vi "UHR-Fleezers Control (host) - 12.7b.vi"() -> ()   [LabVIEW 2012] (continued)
                                frame #0 {
                                n1177 = property on="Trap Delta (MHz)" class="DigNum (strict)"("Val(Sgnl)"=w1735) -> ()  [unwired: 2 in, 2 out]
                                }
                                frame #1 {
                                n1178 = Wait (ms)(milliseconds to wait=u32 500) -> ()  [unwired: 1 out]
                                }
                                frame #2 {
                                n1179 = local read "Shift confocal"() -> (w1739:bool)
                                n1180 = local read "Mean"() -> (w1737:dbl)
                                n1181 = Greater?(x=w1737, y=11.0) -> (0:w1740:bool)
                                n1182 = Not(x=w1740) -> (.not. x?=w1741:bool)
                                n1183 = And(x=w1741, y=w1739) -> (x .and. y?=w1743:bool)
                                n1184 = And(x=w1740, y=w1739) -> (x .and. y?=w1742:bool)
                                n1185 = case shown="True" w1742 {
                                frame False {
                                }
                                frame True {
                                n1186 = local read "Confocal Y 2 (V)"() -> (w1747:dbl)
                                n1187 = local read "Confocal X 2 (V)"() -> (w1746:dbl)
                                n1188 = property on="AO1" class="Slide (strict)"("Val(Sgnl)"=w1747) -> ()  [unwired: 2 in, 2 out]
                                n1189 = property on="AO2" class="Slide (strict)"("Val(Sgnl)"=w1746) -> ()  [unwired: 2 in, 2 out]
                                }
                                }
                                n1190 = case shown="True" w1743 {
                                frame False {
                                }
                                frame True {
                                n1191 = local read "Confocal X 1 (V)"() -> (w1744:dbl)
                                n1192 = local read "Confocal Y 1 (V)"() -> (w1745:dbl)
                                n1193 = property on="AO2" class="Slide (strict)"("Val(Sgnl)"=w1744) -> ()  [unwired: 2 in, 2 out]
                                n1194 = property on="AO1" class="Slide (strict)"("Val(Sgnl)"=w1745) -> ()  [unwired: 2 in, 2 out]
                                }
                                }
                                }
                                }
                                }
                                }
                                }
                              }
                            }
                          }
                          n1195 = local read "Time (s)"() -> (w1681:dbl)
                          "Fl. High" <- TRUE ("Yanking")
                        }
                        frame #1 {
                          n1196 = local read "Auto F Reset"() -> (w1748:bool)
                          n1197 = case shown="True" w1748 {
                            tunnel: w1753 -> [_ w1757]
                            tunnel: w1752 -> [_ w1756]
                            tunnel: w1751 -> [_ w1755]
                            tunnel: w1749 -> [_ w1754]
                            frame False {
                            }
                            frame True {
                              n1198 = node-c288() -> (w1759:T23)  [unwired: 4 out]
                              n1199 = timed-loop {
                                timing: w1759 -> [_]
                                timing-out: [_] -> w1758
                                tunnel: w1757 -> [w1777]
                                tunnel: w1756 -> [w1776]
                                tunnel: w1755 -> [w1775]
                                tunnel: w1754 -> [w1774]
                                stop <- w1760 stop-if-true
                                n1200 = node-c288() -> ()  [unwired: 2 out]
                                n1201 = local read "Fl. Delta Thresh. (kHz)"() -> (w1768:dbl)
                                n1202 = local read "Fl. Triggered..."() -> (w1773:bool)
                                n1203 = local read "Delta Fl. 1"() -> (w1764:dbl)
                                n1204 = local read "Delta Fl. 2"() -> (w1762:dbl)
                                n1205 = local read "Stop All"() -> (w1771:bool)
                                n1206 = local read "APD to Watch"() -> (w1763:bool)
                                n1207 = Select(t=w1764, s=w1763, f=w1762) -> (s? t:f=w1761:dbl)
                                n1208 = Not(x=w1773) -> (.not. x?=w1772:bool)
                                n1209 = Multiply(x=w1768, y=1000.0) -> (x*y=w1767:dbl)
                                n1210 = Negate(x=w1767) -> (-x=w1766:dbl)
                                n1211 = Less?(x=w1761, y=w1766) -> (x < y?=w1770:bool)
                                n1212 = Compound Arithmetic op=OR(w1770, w1771, w1772, "Reset Force") -> (w1760:bool)
                                n1213 = case shown="True" w1760 {
                                tunnel: w1777 -> [_ w1792]
                                tunnel: w1776 -> [_ w1791]
                                tunnel: w1775 -> [_ w1781]
                                tunnel: w1774 -> [_ w1783]
                                frame False {
                                }
                                frame True {
                                n1214 = local read "Time (s)"() -> (w1782:dbl)
                                n1215 = case shown="\"Yank\"" w1791 {
                                tunnel: w1792 -> [_ w1795]
                                tunnel: w1783 -> [_ w1793]
                                frame "Image", Default {
                                }
                                frame "Yank" {
                                n1216 = flat-sequence {
                                tunnel: [w1801] -> w1796
                                tunnel: w1795 -> [w1801]
                                tunnel: [w1797] -> w1794
                                tunnel: w1793 -> [w1797]
                                tunnel: w1796 -> [w1804]
                                tunnel: w1794 -> [w1802]
                                frame #0 {
                                n1217 = local read "Yank Delay (s)"() -> (w1800:dbl)
                                n1218 = Multiply(x=w1800, y=1000.0) -> (x*y=w1798:dbl)
                                n1219 = Wait (ms)(milliseconds to wait=w1798) -> ()  [unwired: 1 out]
                                }
                                frame #1 {
                                n1220 = local read "Yank to which?"() -> (w1803:bool)
                                n1221 = case shown="False" w1803 {
                                tunnel: w1804 -> [_ w1831]
                                tunnel: w1802 -> [w1805 _]
                                frame False {
                                n1222 = flat-sequence {
                                tunnel: w1805 -> [w1806]
                                frame #0 {
                                n1223 = property on="Trap Pos FB SP" class="DigNum (strict)"("Val(Sgnl)"=w1806) -> ()  [unwired: 2 in, 2 out]
                                }
                                frame #1 {
                                n1224 = Wait (ms)(milliseconds to wait=u32 700) -> ()  [unwired: 1 out]
                                }
                                frame #2 {
                                n1225 = local read "Action (%)"() -> (w1811:dbl)
                                n1226 = Absolute Value(x=w1811) -> (abs(x)=w1810:dbl)
                                n1227 = Greater?(x=w1810, y=70.0) -> (0:w1808:bool)
                                n1228 = property on="Remove Action Offset" class="Bool (strict)"("Val(Sgnl)"=w1808) -> ()  [unwired: 2 in, 2 out]
                                }
                                frame #3 {
                                n1229 = for {
                                N: 4 -> [_]
                                n1230 = flat-sequence {
                                frame #0 {
                                n1231 = Wait (ms)(milliseconds to wait=u32 500) -> ()  [unwired: 1 out]
                                }
                                frame #1 {
                                n1232 = local read "Action (%)"() -> (w1817:dbl)
                                n1233 = Absolute Value(x=w1817) -> (abs(x)=w1816:dbl)
                                n1234 = Greater?(x=w1816, y=70.0) -> (0:w1814:bool)
                                n1235 = property on="Remove Action Offset" class="Bool (strict)"("Val(Sgnl)"=w1814) -> ()  [unwired: 2 in, 2 out]
                                }
                                }
                                }
                                }
                                frame #4 {
                                n1236 = local read "Shift confocal"() -> (w1822:bool)
                                n1237 = local read "Mean"() -> (w1824:dbl)
                                n1238 = Greater?(x=w1824, y=11.0) -> (0:w1821:bool)
                                n1239 = Not(x=w1821) -> (.not. x?=w1820:bool)
                                n1240 = And(x=w1821, y=w1822) -> (x .and. y?=w1819:bool)
                                n1241 = And(x=w1820, y=w1822) -> (x .and. y?=w1818:bool)
                                n1242 = case shown="True" w1819 {
                                frame False {
                                }
                                frame True {
                                n1243 = local read "Confocal Y 2 (V)"() -> (w1828:dbl)
                                n1244 = local read "Confocal X 2 (V)"() -> (w1827:dbl)
                                n1245 = property on="AO2" class="Slide (strict)"("Val(Sgnl)"=w1827) -> ()  [unwired: 2 in, 2 out]
                                n1246 = property on="AO1" class="Slide (strict)"("Val(Sgnl)"=w1828) -> ()  [unwired: 2 in, 2 out]
                                }
                                }
                                n1247 = case shown="True" w1818 {
                                frame False {
                                }
                                frame True {
                                n1248 = local read "Confocal X 1 (V)"() -> (w1825:dbl)
                                n1249 = local read "Confocal Y 1 (V)"() -> (w1826:dbl)
                                n1250 = property on="AO1" class="Slide (strict)"("Val(Sgnl)"=w1826) -> ()  [unwired: 2 in, 2 out]
                                n1251 = property on="AO2" class="Slide (strict)"("Val(Sgnl)"=w1825) -> ()  [unwired: 2 in, 2 out]
                                }
                                }
                                }
                                frame #5 {
                                n1252 = Wait (ms)(milliseconds to wait=u32 1500) -> ()  [unwired: 1 out]
                                }
                                frame #6 {
                                n1253 = property on="Rem fb disp offset" class="Bool (strict)"("Val(Sgnl)"=TRUE ("Value (Signaling)")) -> ()  [unwired: 2 in, 2 out]
                                }
                                }
                                }
                                frame True {
                                n1254 = flat-sequence {
                                tunnel: w1831 -> [w1832]
                                frame #0 {
                                n1255 = property on="Trap Delta (MHz)" class="DigNum (strict)"("Val(Sgnl)"=w1832) -> ()  [unwired: 2 in, 2 out]
                                }
                                frame #1 {
                                n1256 = Wait (ms)(milliseconds to wait=u32 500) -> ()  [unwired: 1 out]
                                }
                                frame #2 {
                                n1257 = local read "Shift confocal"() -> (w1838:bool)
                                n1258 = local read "Mean"() -> (w1840:dbl)
                                n1259 = Greater?(x=w1840, y=11.0) -> (0:w1837:bool)
                                n1260 = Not(x=w1837) -> (.not. x?=w1836:bool)
                                n1261 = And(x=w1837, y=w1838) -> (x .and. y?=w1835:bool)
                                n1262 = And(x=w1836, y=w1838) -> (x .and. y?=w1834:bool)
                                n1263 = case shown="True" w1835 {
                                frame False {
                                }
                                frame True {
                                n1264 = local read "Confocal Y 2 (V)"() -> (w1844:dbl)
                                n1265 = local read "Confocal X 2 (V)"() -> (w1843:dbl)
                                n1266 = property on="AO2" class="Slide (strict)"("Val(Sgnl)"=w1843) -> ()  [unwired: 2 in, 2 out]
                                n1267 = property on="AO1" class="Slide (strict)"("Val(Sgnl)"=w1844) -> ()  [unwired: 2 in, 2 out]
                                }
                                }
                                n1268 = case shown="True" w1834 {
                                frame False {
                                }
                                frame True {
                                n1269 = local read "Confocal Y 1 (V)"() -> (w1842:dbl)
                                n1270 = local read "Confocal X 1 (V)"() -> (w1841:dbl)
                                n1271 = property on="AO2" class="Slide (strict)"("Val(Sgnl)"=w1841) -> ()  [unwired: 2 in, 2 out]
                                n1272 = property on="AO1" class="Slide (strict)"("Val(Sgnl)"=w1842) -> ()  [unwired: 2 in, 2 out]
                                }
                                }
                                }
                                }
                                }
                                }
                                }
                                }
                                }
                                }
                                n1273 = local read "Messages"() -> (w1790:string)
                                n1274 = Subtract(x=w1782, y=w1781) -> (x-y=w1788:dbl)
                                "Duration (s)" <- w1788
                                n1275 = Number To Decimal String(number=w1788, width (-)=i16 0) -> (decimal integer string=w1786:string)
                                n1276 = Concatenate Strings(w1786, " s fluorescence event." ("string")) -> (w1784:string)
                                n1277 = call "Update messages.vi"("Message to add"=w1784, "Old message string"=w1790) -> ("New message string"=w1789:string)
                                n1278 = local write "Reset Force"(FALSE ("Reset Force")) -> ()
                                n1279 = local write "Waiting"(TRUE ("Waiting")) -> ()
                                n1280 = local write "Messages"(w1789) -> ()
                                n1281 = local write "Fl. High"(FALSE ("Fl. High")) -> ()
                                n1282 = call <vilib>:"Beep.vi"() -> ()  [unwired: 3 in, 9 out]
                                }
                                }
                                n1283 = node-c288() -> ()  [unwired: 2 out]
                              }
                              n1284 = node-c288(w1758) -> ()  [unwired: 1 out]
                            }
                          }
                        }
                      }
                      n1285 = local read "Trap Delta (MHz)"() -> (w1673:dbl)
                      n1286 = local read "Trap Pos FB SP"() -> (w1668:fxp<+/-,16,1>)
                    }
                  }
                }
                frame #1 {
                  n1287 = local read "Stop All"() -> (w1854:bool)
                  n1288 = local read "Fl. Triggered..."() -> (w1852:bool)
                  n1289 = Not(x=w1852) -> (.not. x?=w1853:bool)
                  n1290 = Or(x=w1853, y=w1854) -> (x .or. y?=w1851:bool)
                }
              }
              n1291 = case shown="True" w1445 {
                frame False {
                }
                frame True {
                  n1292 = local read "Confocal Y 1 (V)"() -> (w1455:dbl)
                  n1293 = local read "Confocal X 1 (V)"() -> (w1454:dbl)
                  n1294 = property on="AO2" class="Slide (strict)"("Val(Sgnl)"=w1454) -> ()  [unwired: 2 in, 2 out]
                  n1295 = property on="AO1" class="Slide (strict)"("Val(Sgnl)"=w1455) -> ()  [unwired: 2 in, 2 out]
                }
              }
              n1296 = case shown="True" w1445 {
                frame False {
                }
                frame True {
                  w1453 = FALSE ("Fl. High")
                  n1297 = local write "Waiting"(w1453) -> ()
                  n1298 = local write "Fl. High"(w1453) -> ()
                }
              }
              n1299 = node-c288() -> ()  [unwired: 2 out]
            }
            n1300 = node-c288(w1443) -> ()  [unwired: 1 out]
          }
        }
      }
      event "Stop All": Value Change {
        n1301 = event-data() -> ()  [unwired: 7 out]
        n1302 = local read "Stop All"() -> (w1859:bool)
      }
    }
    n1303 = node-c288() -> ()  [unwired: 2 out]
  }
  n1304 = timed-loop "Basic control parameters (all FPGA settings, other basic controls)" {
    tunnel: w23 -> [w1868]
    shift-right: [w1867] -> _
    shift-left: errorcluster {"status"=FALSE, "code"=0, "source"=""} ("error out") -> [w1866]
    tunnel: [w1865] -> _
    timing: w133 -> [_]
    timing-out: [_] -> w132
    tunnel: w106 -> [w1864]
    tunnel: w78 -> [w1863]
    tunnel: w77 -> [w1862]
    tunnel: w76 -> [w1861]
    tunnel: w75 -> [w1860]
    stop <- w1865 stop-if-true
    n1305 = node-c288() -> ()  [unwired: 2 out]
    n1306 = event shown="[14] \"DIO count 1 (ticks)\", \"DIO count 2 (ticks)\", \"DIO count 3 (ticks)\", \"Interlace\", \"Number Interlace Sets\", \"Not-Interlacing Set\", \"BD 1 Delay (ticks)\", \"BD 2 Delay (Ticks)\", \"Next trap write delay (ticks)\", \"XY phase ext loop method\", \"Amp switch delay 2\", \"BD 2 Delay (Ticks) 2\", \"BD 1 Delay (ticks) 2\": Value Change" {
      selector: _ -> [_ _ _ _ _ _ _ _ _ _ _ _ _ _ _ _ _ _ _ _ _ _ _ _ _ _ _ _ _ _ _ _ _ _ _ _ _ _ _ _ _ _ _ _ _ _ _ _ _ _ _ _ _ _ _ _ _ _ _ _ _ _ _ _ _ _ _ _ _ _ _ _ _ _]
      dyn-events: _ -> [_ _ _ _ _ _ _ _ _ _ _ _ _ _ _ _ _ _ _ _ _ _ _ _ _ _ _ _ _ _ _ _ _ _ _ _ _ _ _ _ _ _ _ _ _ _ _ _ _ _ _ _ _ _ _ _ _ _ _ _ _ _ _ _ _ _ _ _ _ _ _ _ _ _]
      timeout: _ -> [_ _ _ _ _ _ _ _ _ _ _ _ _ _ _ _ _ _ _ _ _ _ _ _ _ _ _ _ _ _ _ _ _ _ _ _ _ _ _ _ _ _ _ _ _ _ _ _ _ _ _ _ _ _ _ _ _ _ _ _ _ _ _ _ _ _ _ _ _ _ _ _ _ _]
      tunnel: w1868 -> [w1909 _ _ _ w1947 _ w1969 _ _ _ _ w2035 _ _ w2085 w2091 w2098 w2103 w2176 _ w2192 w2217 w2238 w2259 w2279 w2308 w2334 w2337 w2341 w2436 w2441 w2479 _ w2514 w2518 w2529 w2533 w2537 _ w2545 _ _ _ _ _ _ _ _ _ _ _ _ _ _ _ _ _ w2923 _ w2940 _ w2947 w2965 _ w2972 w2980 w2995 w3011 w3017 _ w3026 _ w3045 _]
      tunnel: [w1908 _ _ _ w1937 _ w1968 _ _ w2000 _ w2014 _ _ w2084 w2087 w2097 w2100 w2170 _ w2191 w2216 w2236 w2257 w2277 w2302 w2332 _ w2339 w2434 w2439 w2477 _ w2512 w2516 w2520 w2531 w2535 _ w2543 _ _ _ _ _ _ _ _ _ _ _ _ _ _ _ _ _ w2921 _ _ _ _ w2962 _ _ _ _ _ _ _ _ _ _ _] -> w1867
      tunnel: w1866 -> [w1907 _ _ _ w1946 _ w1967 _ _ w2000 _ w2034 _ _ w2083 w2086 w2096 w2099 w2175 _ w2190 w2215 w2237 w2258 w2278 w2307 w2333 w2336 w2340 w2435 w2440 w2478 _ w2513 w2517 w2528 w2532 w2536 _ w2544 _ _ _ _ _ _ _ _ _ _ _ _ _ _ _ _ _ w2922 _ w2939 _ w2946 w2964 _ w2971 w2979 w2994 w3010 w3016 _ w3025 _ w3044 _]
      tunnel: [_ _ _ _ _ _ _ _ _ w1999 _ _ _ _ _ _ _ _ _ _ _ _ _ _ _ _ _ _ _ _ _ _ _ _ _ _ _ _ _ _ _ _ _ _ _ _ _ _ _ _ _ _ _ _ _ _ _ _ _ _ _ _ _ _ _ _ _ _ _ _ _ _ _ _] -> w1865
      tunnel: [_ _ _ _ _ _ _ "Round T1 X" _ _ _ _ _ _ _ _ _ _ _ _ _ _ _ _ _ _ _ _ _ _ _ _ _ _ _ _ _ _ _ _ _ _ _ _ _ _ _ _ _ _ _ _ _ _ _ _ _ _ _ _ _ _ _ _ _ _ _ _ _ _ _ _ _ _] -> _
      tunnel: [_ _ _ "Adjust Scale\nto Mean" _ _ _ _ _ _ _ _ _ _ _ _ _ _ _ _ _ _ _ _ _ _ _ _ "Test ttrig" _ _ _ _ _ _ _ _ _ _ _ _ _ _ _ _ _ _ "Flush Sample" "Flush Pump 3" "Flush Pump 1" "Clear Volume" _ _ _ _ _ _ _ _ _ _ _ _ _ _ _ _ _ _ _ _ _ _ _] -> _
      tunnel: [_ _ _ _ _ _ _ _ "Round T2 X" _ "Delayed Interlace Start" _ _ _ _ _ _ _ _ _ _ _ _ _ _ _ _ _ _ _ _ _ _ _ _ _ _ _ _ _ _ _ _ _ _ _ _ _ _ _ _ _ _ _ _ _ _ _ _ _ _ _ _ _ _ _ _ _ _ _ _ _ _ _] -> _
      tunnel: w1864 -> [_ _ _ _ _ _ _ _ _ _ _ _ _ _ _ _ _ _ _ _ _ _ _ _ _ _ _ _ _ _ _ _ _ _ _ _ _ _ _ _ _ _ _ w2702 w2709 w2716 w2721 w2730 _ _ w2836 _ _ _ _ _ _ _ _ _ _ _ _ _ _ _ _ _ _ _ _ _ _ _]
      tunnel: w1863 -> [_ _ _ _ _ _ _ _ _ _ _ _ _ _ _ _ _ _ _ _ _ _ _ _ _ _ _ _ _ _ _ _ _ _ _ _ _ _ _ _ _ w2619 _ _ _ _ _ _ w2774 _ _ w2842 _ w2851 _ w2865 _ _ _ _ _ _ _ _ _ _ _ _ _ _ _ _ _ _]
      tunnel: w1862 -> [_ _ _ _ _ _ _ _ _ _ _ _ _ _ _ _ _ _ _ _ _ _ _ _ _ _ _ _ _ _ _ _ _ _ _ _ _ _ _ _ _ _ _ _ _ _ _ _ _ _ _ _ _ _ _ _ _ _ _ _ _ _ _ _ _ _ _ _ _ _ _ _ _ _]
      tunnel: w1861 -> [_ _ _ _ _ _ _ _ _ _ _ _ _ _ _ _ _ _ _ _ _ _ _ _ _ _ _ _ _ _ _ _ _ _ _ _ _ _ _ _ w2556 _ _ _ _ _ _ _ _ w2804 _ _ w2847 _ w2858 _ w2890 _ _ _ _ _ _ _ _ _ _ _ _ _ _ _ _ _]
      tunnel: w1860 -> [_ _ _ _ _ _ _ _ _ _ _ _ _ _ _ _ _ _ _ _ _ _ _ _ _ _ _ _ _ _ _ _ _ _ _ _ _ _ _ _ _ _ _ _ _ _ _ _ _ _ _ _ _ _ _ _ _ _ _ _ _ _ _ _ _ _ _ _ _ _ _ _ _ _]
      event "AI Count (ticks)", "Sets to FIFO (Traps)", "Save ave N", "FPGA Ave.", "# Samples/channel", "N sets to save": Value Change {
        # "So that if 'Save ave N' is updated, the AOD scanning code updates too."
        n1307 = event-data() -> ()  [unwired: 6 out]
        n1308 = local read "AI Count (ticks)"() -> (w1891:u16)
        n1309 = Unbundle By Name("Sets to FIFO (Traps)") -> ("Set 1"=w1874:bool, "Set 2"=w1873:bool, "Set 3"=w1872:bool)
        n1310 = Boolean To (0,1)(Boolean="Sets to FIFO (Traps)") -> (0, 1=w1899:cluster{"Set 1":i16, "Set 2":i16, "Set 3":i16})
        n1311 = xnode "Read/Write Control"("FPGA VI Reference In"=w1909, "error in"=w1907, "ai count"=w1891, "Set 1"=w1874, "Set 2"=w1873, "Set 3"=w1872, "N of AI1 Int Acq Sets"="N Acq Sets (Traps + Fl.)") -> ("error out"=w1908:errorcluster)  [unwired: 1 out]
        n1312 = Cluster To Array(cluster=w1899) -> (array=w1898:i16[])
        n1313 = To Unsigned Long Integer(number=w1898) -> (unsigned 32bit integer=w1880:u32[])
        n1314 = local read "Scan steps (AOD)"() -> (w1900:u64)
        n1315 = Multiply(x=w1891, y="N Acq Sets (Traps + Fl.)") -> (x*y=w1889:u16)
        n1316 = Divide(x=40000000.0, y=w1891) -> (x/y=w1883:dbl)
        "AI rate (Hz)" <- w1883
        "Ave. Rate (Hz)" <- w1883
        n1317 = Add Array Elements(numeric array=w1880) -> (sum=w1892:u32)
        "Trap Sets" <- w1892
        n1318 = Reciprocal(x=w1883) -> (1/x=→"Ave. Period (s)":dbl)
        n1319 = property on="Scan steps (AOD)" class="DigNum (strict)"("Val(Sgnl)"=w1900) -> ()  [unwired: 2 in, 2 out]
        n1320 = Divide(x=w1883, y="N Acq Sets (Traps + Fl.)") -> (x/y=w1904:dbl)
        "Data Rate (Hz)" <- w1904
        n1321 = Reciprocal(x=w1904) -> (1/x=→"Data Period (s)":dbl)
        n1322 = local read "Save ave N"() -> (w1903:dbl)
        n1323 = Divide(x=w1904, y=w1903) -> (x/y=w1902:dbl)
        "Save Data Rate (Hz)" <- w1902
        n1324 = Reciprocal(x=w1902) -> (1/x=→"Save Data Period (s)":dbl)
        n1325 = Multiply(x=w1889, y="# Samples/trap") -> (x*y=w1887:u32)
        "Counts/DMA" <- w1887
        n1326 = property on="Trap Disp. Downsample" class="DigNum (strict)"("Maximum"="# Samples/trap") -> ()  [unwired: 2 in, 2 out]
        n1327 = Multiply(x=w1892, y="# Samples/trap") -> (x*y=w1881:u32)
        "# Samples/channel" <- w1881
        n1328 = Multiply(x=w1881, y=u32 8) -> (x*y=→"Trap AI Elements/DMA read":u32)
        n1329 = local read "APD Int. Count"() -> (w1888:u32)
        n1330 = Multiply(x=w1881, y=u32 3) -> (x*y=→"Trap Pos Elements/DMA read":u32)
        n1331 = Divide(x=w1887, y=w1888) -> (x/y=w1878:dbl)
        "APD Samples/FIFO Acq." <- w1878
        n1332 = Divide(x=w1887, y=40000000.0) -> (x/y=w1885:dbl)
        "DMA Update Period (s)" <- w1885
        n1333 = local read "Number of APDs"() -> (w1871:u8)
        n1334 = Multiply(x=w1871, y=w1878) -> (x*y=→"APD Elements/DMA read":dbl)
        n1335 = property on="APD Disp. Downsample" class="DigNum (strict)"("Maximum"=w1878) -> ()  [unwired: 2 in, 2 out]
        n1336 = local read "N sets to save"() -> (w1897:u32)
        n1337 = Multiply(x=w1885, y=w1897) -> (x*y=→"Total Time (s)":dbl)
        "FPGA Averaging" <- FALSE ("FPGA Averaging")
      }
      event "Remove Offset": Value Change {
        n1338 = event-data() -> ()  [unwired: 7 out]
        n1339 = local write "Remove Offset"(FALSE ("Remove Offset")) -> ()
        n1340 = local read "Bead Mean (nm)"() -> (w1911:dbl)
        n1341 = local read "Offset (nm)"() -> (w1912:dbl)
        n1342 = Add(x=w1911, y=w1912) -> (x+y=w1910:dbl)
        n1343 = local write "Offset (nm)"(w1910) -> ()
        n1344 = disable-structure shown="Disabled" {
          frame Disabled {
            n1345 = local read "Bead Mean (nm)"() -> (w1917:dbl)
            n1346 = Add(y=w1917) -> (x=w1916:dbl, x+y=w1915:dbl)
            n1347 = Subtract(x=w1917, y=w1916) -> (x-y=w1914:dbl)
            n1348 = property on="Bead Separation" class="WFChart (strict)"("YScale.Minimum"=w1914) -> ()  [unwired: 2 in, 2 out]
            n1349 = property on="Bead Separation" class="WFChart (strict)"("YScale.Maximum"=w1915) -> ()  [unwired: 2 in, 2 out]
          }
          frame Enabled {
          }
        }
      }
      event "Detector Type": Value Change {
        n1350 = event-data() -> ()  [unwired: 7 out]
        n1351 = local read "AI labels"() -> (w1918:string[])
        n1352 = property on="High Res. Display" class="Ring (strict)"("Strings []"=w1918) -> ()  [unwired: 2 in, 2 out]
        n1353 = Build Array (concatenate)(w1918, "none") -> (w1919:string[])
        n1354 = property on="FFT 1 Choice 1" class="Ring (strict)"("Strings []"=w1919) -> ()  [unwired: 2 in, 2 out]
        n1355 = property on="FFT 1 Choice 2" class="Ring (strict)"("Strings []"=w1919) -> ()  [unwired: 2 in, 2 out]
        n1356 = property on="FFT 2 Choice 1" class="Ring (strict)"("Strings []"=w1919) -> ()  [unwired: 2 in, 2 out]
        n1357 = property on="FFT 2 Choice 2" class="Ring (strict)"("Strings []"=w1919) -> ()  [unwired: 2 in, 2 out]
        n1358 = Bundle("APD 1", "APD 2") -> (w1922:cluster{string, string})  [unwired: 1 out]
        n1359 = Cluster To Array(cluster=w1922) -> (array=w1920:string[])
        n1360 = Build Array (concatenate)(w1920, w1919) -> (w1924:string[])
        n1361 = Array Size(array=w1924) -> (size(s)=w1925:i32)
        n1362 = property on="Signals to Plot" class="LstBox (strict)"("Item Names"=w1924) -> ()  [unwired: 2 in, 2 out]
        n1363 = property on="Signals to Plot" class="LstBox (strict)"("Number of Rows"=w1925) -> ()  [unwired: 2 in, 2 out]
        n1364 = property on="All Signals" class="WFChart (strict)"("LegNumRows"=w1925) -> ()  [unwired: 2 in, 2 out]
      }
      event "Adjust Scale\nto Mean": Value Change {
        n1365 = event-data() -> ()  [unwired: 7 out]
        n1366 = local read "APD 1 Rate (Hz)"() -> (w1934:dbl)
        n1367 = Multiply(x=1000.0, y="Above (kHz)") -> (x*y=w1932:dbl)
        n1368 = Multiply(x=1000.0, y="Below (kHz)") -> (x*y=w1930:dbl)
        n1369 = Add(x=w1932, y=w1934) -> (x+y=w1927:dbl)
        n1370 = Subtract(x=w1934, y=w1930) -> (x-y=w1928:dbl)
        n1371 = property on="APD Chart" class="WFChart (strict)"("YScale.Minimum"=w1928) -> ()  [unwired: 2 in, 2 out]
        n1372 = property on="APD Chart" class="WFChart (strict)"("YScale.Maximum"=w1927) -> ()  [unwired: 2 in, 2 out]
      }
      event "Phase adj. (AI1)", "+ phase (AI1)", "- phase (AI1)": Value Change {
        n1373 = event-data() -> ()  [unwired: 7 out]
        n1374 = Negate(x="Phase adj. (AI1)") -> (-x=w1944:i16)
        n1375 = Select(t=w1944, s="- phase (AI1)", f="Phase adj. (AI1)") -> (s? t:f=w1943:i16)
        n1376 = xnode "Read/Write Control"("FPGA VI Reference In"=w1947, "error in"=w1946, "Phase count adjustment"=w1943) -> ("FPGA VI Reference Out"=w1942:T20, "error out"=w1941:errorcluster)  [unwired: 1 in]
        n1377 = Or(x="- phase (AI1)", y="+ phase (AI1)") -> (x .or. y?=w1938:bool)
        n1378 = xnode "Read/Write Control"("FPGA VI Reference In"=w1942, "error in"=w1941, "+ phase"=w1938) -> ("error out"=w1937:errorcluster)  [unwired: 1 in, 1 out]
      }
      event "Signals to Plot": Double Click {
        w1950 = u32 9868950 ("Color Box")
        n1379 = event-data() -> ("Row"=w1952:i32)  [unwired: 9 out]
        n1380 = property on="All Signals" class="WFChart (strict)"("Active Plot"=w1952) -> (error out=w1963:errorcluster)  [unwired: 2 in, 1 out]
        n1381 = property on="All Signals" class="WFChart (strict)" props=["Plot", "Visible?", "Plot", "Plot Color"](error in=w1963) -> (error out=w1962:errorcluster, "Plot.Visible?"=w1961:bool)  [unwired: 1 in, 2 out]
        n1382 = Select(t=FALSE ("Plot.Visible"), s=w1961, f=TRUE ("Plot.Visible")) -> (s? t:f=w1956:bool)
        n1383 = property on="All Signals" class="WFChart (strict)"(error in=w1962, "Plot.Visible?"=w1956) -> (error out=w1958:errorcluster)  [unwired: 1 in, 1 out]
        n1384 = property on="All Signals" class="WFChart (strict)"(error in=w1958) -> (error out=w1953:errorcluster, "Plot.Plot Color"=w1957:u32)  [unwired: 1 in, 1 out]
        n1385 = property on="Signals to Plot" class="LstBox (strict)"(error in=w1953, "Active Row"=w1952) -> (error out=w1951:errorcluster)  [unwired: 1 in, 1 out]
        n1386 = Select(t=w1957, s=w1956, f=u32 0) -> (s? t:f=w1954:u32)
        n1387 = property on="Signals to Plot" class="LstBox (strict)"(error in=w1951, "CellFontColor"=w1954, "SelColor"=w1950, "CellBG"=w1950, "CellFontSize"=u32 20 ("Active Row:Cell Font:Size"), "CellFontBold"=TRUE ("Active Row:Cell Font:Bold")) -> ()  [unwired: 1 in, 2 out]
      }
      event "BD 1 Frequency 1 (MHz)", "BD 1 Frequency 2 (MHz)", "BD 1 Frequency 3 (MHz)", "BD 2 Frequency 1 (MHz)", "BD 2 Frequency 2 (MHz)", "BD 2 Frequency 3 (MHz)", "Trap Delta (MHz)": Value Change {
        n1388 = event-data() -> ("CtlRef"=w1966:refnum<vi>)  [unwired: 6 out]
        n1389 = control-ref of="Trap Delta (MHz)"() -> (w1965:refnum<vi>)
        n1390 = Equal?(x=w1965, y=w1966) -> (x = y?=w1964:bool)
        n1391 = case shown="False" "Oscillate Set 1" {
          tunnel: w1969 -> [w1989 _]
          tunnel: [w1988 w1992] -> w1968
          tunnel: w1967 -> [w1987 w1992]
          tunnel: w1964 -> [w1972 _]
          frame False {
            n1392 = local read "BD 1 Frequency 2 (MHz)"() -> (w1976:dbl)
            n1393 = local read "BD 1 Frequency 1 (MHz)"() -> (w1974:dbl)
            n1394 = Subtract(x=w1976, y="Trap Delta (MHz)") -> (x-y=w1973:dbl)
            n1395 = Select(t=w1973, s=w1972, f=w1974) -> (s? t:f=w1971:dbl)
            n1396 = local read "Y RF Frequency Limits (MHz)"() -> (w1977:T16)
            n1397 = local read "X RF Frequency Limits (MHz)"() -> (w1978:T16)
            n1398 = local read "BD 1 Frequency 3 (MHz)"() -> (w1990:dbl)
            n1399 = local write "BD 1 Frequency 1 (MHz)"(w1971) -> ()
            n1400 = local read "BD 2 Frequency 1 (MHz)"() -> (w1981:dbl)
            n1401 = local read "BD 2 Frequency 2 (MHz)"() -> (w1980:dbl)
            n1402 = local read "BD 2 Frequency 3 (MHz)"() -> (w1991:dbl)
            n1403 = call "set RF board frequency - interlace.vi"("Board 2 Frequency Limits"=w1977, "Board 1 Frequency Limits"=w1978, "error in"=w1987, "FPGA VI Reference In"=w1989, "Board 2 Frequency 3 (MHz)"=w1991, "Board 1 Frequency 3 (MHz)"=w1990, "Board 2 Frequency 2 (MHz)"=w1980, "Board 2 Frequency 1 (MHz)"=w1981, "Board 1 Frequency 2 (MHz)"=w1976, "Board 1 Frequency 1  (MHz)"=w1971) -> ("error out"=w1988:errorcluster)  [unwired: 1 out]
            n1404 = Subtract(x=w1981, y=w1980) -> (x-y=w1985:dbl)
            n1405 = Subtract(x=w1971, y=w1976) -> (x-y=w1986:dbl)
            n1406 = Square(x=w1985) -> (x^2=w1983:dbl)
            n1407 = Square(x=w1986) -> (x^2=w1984:dbl)
            n1408 = Add(x=w1984, y=w1983) -> (x+y=w1982:dbl)
            n1409 = Square Root(x=w1982) -> (sqrt(x)=w1979:dbl)
            n1410 = local write "Trap Delta (MHz)"(w1979) -> ()
            n1411 = property on="Initial delta (MHz)" class="DigNum (strict)"("Val(Sgnl)"=w1979) -> ()  [unwired: 2 in, 2 out]
          }
          frame True {
          }
        }
      }
      event "Round T1 X": Value Change {
        n1412 = event-data() -> ()  [unwired: 7 out]
        n1413 = local read "BD 1 Frequency 1 (MHz)"() -> (w1995:dbl)
        n1414 = Round To Nearest(number=w1995) -> (nearest integer value=w1994:dbl)
        n1415 = property on="BD 1 Frequency 1 (MHz)" class="DigNum (strict)"("Val(Sgnl)"=w1994) -> ()  [unwired: 2 in, 2 out]
      }
      event "Round T2 X": Value Change {
        n1416 = event-data() -> ()  [unwired: 7 out]
        n1417 = local read "BD 1 Frequency 2 (MHz)"() -> (w1997:dbl)
        n1418 = Round To Nearest(number=w1997) -> (nearest integer value=w1996:dbl)
        n1419 = property on="BD 1 Frequency 2 (MHz)" class="DigNum (strict)"("Val(Sgnl)"=w1996) -> ()  [unwired: 2 in, 2 out]
      }
      event "Stop All": Value Change {
        n1420 = event-data() -> ()  [unwired: 7 out]
        n1421 = local read "Stop All"() -> (w1999:bool)
      }
      event "Delayed Interlace Start": Value Change {
        n1422 = event-data() -> ()  [unwired: 7 out]
        n1423 = flat-sequence {
          frame #0 {
            n1424 = Multiply(x="Delay to Interlace (s)", y=1000.0) -> (x*y=w2002:dbl)
            n1425 = Wait (ms)(milliseconds to wait=w2002) -> ()  [unwired: 1 out]
          }
          frame #1 {
            n1426 = property on="Laser interlacing mode" class="RadioBtnsControl (strict)"("Val(Sgnl)"=enum32{"Laser ON", "Laser OFF", "Interlace"}."Interlace" ("Value (Signaling)")) -> ()  [unwired: 2 in, 2 out]
          }
        }
      }
      event "BD 1 Amplitude 1 (%)", "BD 1 Amplitude 2 (%)", "BD 1 Amplitude 3 (%)", "BD 2 Amplitude 1 (%)", "BD 2 Amplitude 2 (%)", "BD 2 Amplitude 3 (%)", "Trap 1 ON", "Trap 2 ON", "Trap 3 ON", "Feedback On/Off", "All FB On/Off": Value Change {
        w2026 = i16 1 ("f")
        n1427 = event-data() -> ()  [unwired: 7 out]
        n1428 = local write "Trap 1 (ON/OFF)"("Trap 1 ON") -> ()
        n1429 = local write "Trap 2 (ON/OFF)"("Trap 2 ON") -> ()
        n1430 = Boolean To (0,1)(Boolean="Trap 3 ON") -> (0, 1=w2027:i16)
        n1431 = Boolean To (0,1)(Boolean="Trap 1 ON") -> (0, 1=w2028:i16)
        n1432 = Boolean To (0,1)(Boolean="Trap 2 ON") -> (0, 1=w2029:i16)
        n1433 = Select(t=w2029, s="Trap ON/OFF X or Y Amp?", f=w2026) -> (s? t:f=w2024:i16)
        n1434 = Select(t=w2028, s="Trap ON/OFF X or Y Amp?", f=w2026) -> (s? t:f=w2025:i16)
        n1435 = Select(t=w2027, s="Trap ON/OFF X or Y Amp?", f=w2026) -> (s? t:f=w2023:i16)
        n1436 = Select(t=w2026, s="Trap ON/OFF X or Y Amp?", f=w2029) -> (s? t:f=w2021:i16)
        n1437 = Select(t=w2026, s="Trap ON/OFF X or Y Amp?", f=w2028) -> (s? t:f=w2022:i16)
        n1438 = Select(t=w2026, s="Trap ON/OFF X or Y Amp?", f=w2027) -> (s? t:f=w2020:i16)
        n1439 = And(x="All FB On/Off", y="Feedback On/Off") -> (x .and. y?=w2018:cluster{"Set 1":bool, "Set 2":bool})
        n1440 = local read "BD 1 Amplitude 1 (%)"() -> (w2038:dbl)
        n1441 = local read "BD 1 Amplitude 2 (%)"() -> (w2037:dbl)
        n1442 = local read "BD 1 Amplitude 3 (%)"() -> (w2036:dbl)
        n1443 = Unbundle By Name(w2018) -> ("Set 1"=w2013:bool, "Set 2"=w2010:bool)
        n1444 = local read "Y RF Amplitude Limits (%)"() -> (w2006:T16)
        n1445 = local read "X RF Amplitude Limits (%)"() -> (w2007:T16)
        n1446 = local read "BD 2 Amplitude 1 (%)"() -> (w2039:dbl)
        n1447 = local read "BD 2 Amplitude 2 (%)"() -> (w2040:dbl)
        n1448 = local read "BD 2 Amplitude 3 (%)"() -> (w2041:dbl)
        n1449 = And(x="Trap 2 ON", y=w2010) -> (x .and. y?=w2008:bool)
        n1450 = And(x="Trap 1 ON", y=w2013) -> (x .and. y?=w2011:bool)
        n1451 = Multiply(x=w2025, y=w2038) -> (x*y=w2033:dbl)
        n1452 = Multiply(x=w2037, y=w2024) -> (x*y=w2031:dbl)
        n1453 = Multiply(x=w2036, y=w2023) -> (x*y=w2032:dbl)
        n1454 = Multiply(x=w2039, y=w2022) -> (x*y=w2042:dbl)
        n1455 = Multiply(x=w2040, y=w2021) -> (x*y=w2043:dbl)
        n1456 = Multiply(x=w2041, y=w2020) -> (x*y=w2044:dbl)
        n1457 = call "set RF board amplitude - interlace.vi"("Board 2 Amplitude Limits"=w2006, "Board 1 Amplitude Limits"=w2007, "error in"=w2034, "FPGA VI Reference In"=w2035, "Board 2 Amplitude 3 (%)"=w2044, "Board 1 Amplitude 3 (%)"=w2032, "Board 2 Amplitude 2 (%)"=w2043, "Board 2 Amplitude 1 (%)"=w2042, "Board 1 Amplitude 2 (%)"=w2031, "Board 1 Amplitude 1 (%)"=w2033) -> ("error out"=w2015:errorcluster, "FPGA VI Reference Out"=w2016:T20)
        n1458 = xnode "Read/Write Control"("FPGA VI Reference In"=w2016, "error in"=w2015, "FB On/Off Set 1"=w2011, "FB On/Off Set 2"=w2008) -> ("error out"=w2014:errorcluster)  [unwired: 1 out]
      }
      event "Load parameters": Value Change {
        n1459 = event-data() -> ()  [unwired: 7 out]
        n1460 = property on="Saved AOD Raster Scan Parameter Sets" class="Arr (strict)"() -> ("Index Values"=w2055:u32[])  [unwired: 2 in, 2 out]
        n1461 = Index Array(array=w2055, index=0) -> (element=w2052:u32)
        n1462 = local write "Load parameters"(FALSE ("Load parameters")) -> ()
        n1463 = Index Array(array="Saved AOD Raster Scan Parameter Sets", index=w2052) -> (element=w2051:T30)
        n1464 = Unbundle By Name(w2051) -> ("Scan Range AOD (nm) 2"=w2050:dbl, "Step Size AOD (nm) 2"=w2049:dbl, "Scan Speed AOD (nm/s) 2"=w2048:dbl, "Number of scans (AOD) 2"=w2047:u16)
        n1465 = flat-sequence {
          tunnel: w2050 -> [w2058]
          tunnel: w2049 -> [w2057]
          tunnel: w2048 -> [w2056]
          tunnel: w2047 -> [w2059]
          frame #0 {
            n1466 = local write "Scan Speed (nm/s)"(w2056) -> ()
            n1467 = local write "Scan Range (nm)"(w2058) -> ()
            n1468 = local write "Step Size (nm)"(w2057) -> ()
          }
          frame #1 {
            n1469 = property on="Number of F/B Scans (AOD)" class="DigNum (strict)"("Val(Sgnl)"=w2059) -> ()  [unwired: 2 in, 2 out]
          }
        }
      }
      event "Trap 1 (ON/OFF)", "Trap 2 (ON/OFF)": Value Change {
        n1470 = event-data() -> ()  [unwired: 7 out]
        n1471 = property on="Trap 2 ON" class="Bool (strict)"("Val(Sgnl)"="Trap 2 (ON/OFF)") -> ()  [unwired: 2 in, 2 out]
        n1472 = property on="Trap 1 ON" class="Bool (strict)"("Val(Sgnl)"="Trap 1 (ON/OFF)") -> ()  [unwired: 2 in, 2 out]
      }
      event "DIO count 1 (ticks)", "DIO count 2 (ticks)", "DIO count 3 (ticks)", "Interlace", "Number Interlace Sets", "Not-Interlacing Set", "BD 1 Delay (ticks)", "BD 2 Delay (Ticks)", "Next trap write delay (ticks)", "XY phase ext loop method", "Amp switch delay 2", "BD 2 Delay (Ticks) 2", "BD 1 Delay (ticks) 2": Value Change {
        n1473 = event-data() -> ()  [unwired: 7 out]
        n1474 = local read "DIO count 3 (ticks)"() -> (w2079:u16)
        n1475 = local read "DIO count 1 (ticks)"() -> (w2081:u16)
        n1476 = local read "DIO count 2 (ticks)"() -> (w2080:u16)
        n1477 = To Unsigned Byte Integer(number="Not-Interlacing Set") -> (unsigned 8bit integer=w2070:u8)
        n1478 = Add(x=w2070, y=u8 1) -> (x+y=w2074:u8)
        n1479 = xnode "Read/Write Control"("FPGA VI Reference In"=w2085, "error in"=w2083, "DIO count 1 (ticks)"=w2081, "DIO count 2 (ticks)"=w2080, "DIO count 3 (ticks)"=w2079, "Interlace ON/OFF"="Interlace", "Number Interlace Cycles"="Number Interlace Sets", "Interlace Off Parameters"=w2074, "BD 1 Delay (ticks)"="BD 1 Delay (ticks)", "BD 2 Delay (Ticks)"="BD 2 Delay (Ticks)", "Next trap write delay (ticks)"="Next trap write delay (ticks)", "XY phase ext loop method"="XY phase ext loop method", "Amp switch delay 2"="Amp switch delay 2", "BD 2 Delay (Ticks) 2"="BD 2 Delay (Ticks) 2", "BD 1 Delay (ticks) 2"="BD 1 Delay (ticks) 2") -> ("error out"=w2084:errorcluster)  [unwired: 1 out]
        n1480 = Build Array(w2081, w2080, w2079) -> (w2072:u16[])
        n1481 = Split 1D Array(array=w2072, index="Number Interlace Sets") -> (first subarray=w2082:u16[])  [unwired: 1 out]
        n1482 = Index Array(array=w2072, index=w2070) -> (element=w2071:u16)
        n1483 = Add Array Elements(numeric array=w2082) -> (sum=w2076:u16)
        n1484 = Select(t=w2076, s="Interlace", f=w2071) -> (s? t:f=→"Total Counts (ticks)":u16)
      }
      event "Reset Feedback": Value Change {
        n1485 = event-data() -> ()  [unwired: 7 out]
        n1486 = Unbundle By Name("Reset Feedback") -> ("Set 1"=w2089:bool, "Set 2"=w2088:bool)
        n1487 = xnode "Read/Write Control"("FPGA VI Reference In"=w2091, "error in"=w2086, "FB Reset Set 1"=w2089, "FB Reset Set 2"=w2088) -> ("error out"=w2087:errorcluster)  [unwired: 1 out]
      }
      event "Trap Intensity PID Gains": Value Change {
        n1488 = event-data() -> ()  [unwired: 7 out]
        n1489 = Unbundle By Name("Trap Intensity PID Gains") -> ("proportional gain (Kc)"=w2094:i16, "integral gain (Kc*Ts/Ti)"=w2093:i16, "derivative gain (Kc*Td/Ts)"=w2092:i16)
        n1490 = xnode "Read/Write Control"("FPGA VI Reference In"=w2098, "error in"=w2096, "P1"=w2094, "I1"=w2093, "D1"=w2092) -> ("error out"=w2097:errorcluster)  [unwired: 1 out]
      }
      event "AI2 to Setpoint", "Setpoints (V)": Value Change {
        n1491 = event-data() -> ()  [unwired: 7 out]
        n1492 = xnode "Read/Write Control"("FPGA VI Reference In"=w2103, "error in"=w2099) -> ("FPGA VI Reference Out"=w2102:T20, "error out"=w2101:errorcluster, "AI2 Y Sum Set 1"=w2110:i16, "AI2 Y Sum Set 2"=w2109:i16)
        n1493 = Cluster To Array(cluster="AI2 to Setpoint") -> (array=w2113:bool[])
        n1494 = local read "AI2 (V)"() -> (w2111:cluster{"Set 1":dbl, "Set 2":dbl})
        n1495 = Or Array Elements(Boolean array=w2113) -> (logical OR=w2114:bool)
        n1496 = Bundle By Name(cluster=w2111, "Set 1"=w2110, "Set 2"=w2109) -> (w2108:cluster{"Set 1":dbl, "Set 2":dbl})
        n1497 = Divide(x=w2108, y=3276.7) -> (x/y=w2107:cluster{"Set 1":dbl, "Set 2":dbl})
        "AI2 (V)" <- w2107
        n1498 = case shown="True" w2114 {
          tunnel: [w2117 w2134] -> w2106
          tunnel: "AI2 to Setpoint" -> [_ w2130]
          tunnel: "Setpoints (V)" -> [w2118 w2133]
          tunnel: w2107 -> [_ w2127]
          frame False {
            n1499 = Multiply(x=3276.7, y=w2118) -> (x*y=w2119:cluster{"Set 1":dbl, "Set 2":dbl})
            n1500 = To Word Integer(number=w2119) -> (16bit integer=w2117:cluster{"Set 1":i16, "Set 2":i16})
          }
          frame True {
            n1501 = Unbundle By Name(w2127) -> ("Set 1"=w2126:dbl, "Set 2"=w2125:dbl)
            n1502 = Unbundle By Name(w2133) -> ("Set 1"=w2132:dbl, "Set 2"=w2131:dbl)
            n1503 = Unbundle By Name(w2130) -> ("Set 1"=w2129:bool, "Set 2"=w2128:bool)
            n1504 = Select(t=w2126, s=w2129, f=w2132) -> (s? t:f=w2124:dbl)
            n1505 = Select(t=w2125, s=w2128, f=w2131) -> (s? t:f=w2123:dbl)
            n1506 = Bundle By Name(cluster=w2133, "Set 1"=w2124, "Set 2"=w2123) -> (w2121:cluster{"Set 1":dbl, "Set 2":dbl})
            n1507 = local write "Setpoints (V)"(w2121) -> ()
            n1508 = Multiply(x=3276.7, y=w2121) -> (x*y=w2122:cluster{"Set 1":dbl, "Set 2":dbl})
            n1509 = To Word Integer(number=w2122) -> (16bit integer=w2134:cluster{"Set 1":i16, "Set 2":i16})
          }
        }
        n1510 = Unbundle By Name(w2106) -> ("Set 1"=w2105:i16, "Set 2"=w2104:i16)
        n1511 = xnode "Read/Write Control"("FPGA VI Reference In"=w2102, "error in"=w2101, "FB Setpoint Set 1"=w2105, "FB Setpoint Set 2"=w2104) -> ("error out"=w2100:errorcluster)  [unwired: 1 out]
      }
      event "+ phase (GI)", "- phase (GI)", "+ phase (GI) 2", "- phase (GI) 2", "+ phase (RI)", "- phase (RI)", "+ phase (Green FB)", "- phase (Green FB)": Value Change {
        n1512 = event-data() -> ()  [unwired: 7 out]
        n1513 = Or(x="+ phase (GI)", y="- phase (GI)") -> (x .or. y?=w2169:bool)
        n1514 = Negate(x="Phase adj. (GI)") -> (-x=w2174:i16)
        n1515 = Select(t=w2174, s="+ phase (GI)", f="Phase adj. (GI)") -> (s? t:f=w2173:i16)
        n1516 = Or(x="+ phase (GI) 2", y="- phase (GI) 2") -> (x .or. y?=w2160:bool)
        n1517 = Negate(x="Phase adj. (GI) 2") -> (-x=w2165:i16)
        n1518 = Select(t=w2165, s="+ phase (GI) 2", f="Phase adj. (GI) 2") -> (s? t:f=w2161:i16)
        n1519 = Negate(x="Phase adj. (RI)") -> (-x=w2159:i16)
        n1520 = Or(x="+ phase (RI)", y="- phase (RI)") -> (x .or. y?=w2155:bool)
        n1521 = Select(t=w2159, s="+ phase (RI)", f="Phase adj. (RI)") -> (s? t:f=w2154:i16)
        n1522 = Or(x="+ phase (Green FB)", y="- phase (Green FB)") -> (x .or. y?=w2148:bool)
        n1523 = Negate(x="Phase adj. (Green FB)") -> (-x=w2153:i16)
        n1524 = Select(t=w2153, s="+ phase (Green FB)", f="Phase adj. (Green FB)") -> (s? t:f=w2149:i16)
        n1525 = Negate(x="Phase adj. (BI AO)") -> (-x=w2147:i16)
        n1526 = Or(x="+ phase (BI AO)", y="- phase (BI AO)") -> (x .or. y?=w2137:bool)
        n1527 = Select(t=w2147, s="+ phase (BI AO)", f="Phase adj. (BI AO)") -> (s? t:f=w2139:i16)
        n1528 = Negate(x="Phase adj. (BI DO)") -> (-x=w2143:i16)
        n1529 = Or(x="+ phase (BI DO)", y="- phase (BI DO)") -> (x .or. y?=w2136:bool)
        n1530 = Select(t=w2143, s="+ phase (BI DO)", f="Phase adj. (BI DO)") -> (s? t:f=w2138:i16)
        n1531 = xnode "Read/Write Control"("FPGA VI Reference In"=w2176, "error in"=w2175, "Phase count adjustment (GI)"=w2173, "Phase count adjustment (GI) 2"=w2161, "Phase count adjustment (RI)"=w2154, "Phase count adjustment (Green FB)"=w2149, "Phase count adjustment (BI AO)"=w2139, "Phase count adjustment (BI D)"=w2138) -> ("FPGA VI Reference Out"=w2171:T20, "error out"=w2172:errorcluster)
        n1532 = xnode "Read/Write Control"("FPGA VI Reference In"=w2171, "error in"=w2172, "+ phase (GI)"=w2169, "+ phase (GI) 2"=w2160, "+ phase (RI)"=w2155, "+ phase (Green FB)"=w2148, "+ phase (BI AO)"=w2137, "+ phase (BI D)"=w2136) -> ("error out"=w2170:errorcluster)  [unwired: 1 out]
      }
      event "Green Laser ON/OFF", "Red Laser ON/OFF", "Blue Laser ON/OFF": Value Change {
        # "This loop shouldn't be initialized.  The main 'laser ON' settings should dominate and set the others."
        n1533 = event-data() -> ()  [unwired: 7 out]
        n1534 = property on="Red Laser ON" class="Bool (strict)"("Val(Sgnl)"="Red Laser ON/OFF") -> ()  [unwired: 2 in, 2 out]
        n1535 = property on="Blue Laser ON" class="Bool (strict)"("Val(Sgnl)"="Blue Laser ON/OFF") -> ()  [unwired: 2 in, 2 out]
        n1536 = property on="Green Laser ON" class="Bool (strict)"("Val(Sgnl)"="Green Laser ON/OFF") -> ()  [unwired: 2 in, 2 out]
      }
      event "Laser interlacing mode", "Green Laser ON", "Red Laser ON", "Blue Laser ON": Value Change {
        n1537 = event-data() -> ()  [unwired: 7 out]
        n1538 = local write "Green Laser ON/OFF"("Green Laser ON") -> ()
        n1539 = local write "Blue Laser ON/OFF"("Blue Laser ON") -> ()
        n1540 = local write "Red Laser ON/OFF"("Red Laser ON") -> ()
        n1541 = case shown="True" "Green Laser ON" {
          tunnel: "Laser interlacing mode" -> [_ w2213]
          tunnel: [enum32{"Laser ON", "Laser OFF", "Interlace"}."Laser OFF" ("Green laser mode") w2213] -> w2189
          tunnel: [FALSE w2209] -> w2188
          frame False {
          }
          frame True {
            n1542 = local read "Green FB On/Off"() -> (w2210:bool)
            n1543 = Equal?(x=w2213, y=enum32{"Laser ON", "Laser OFF", "Interlace"}."Interlace") -> (x = y?=w2211:bool)
            n1544 = And(x=w2211, y=w2210) -> (x .and. y?=w2209:bool)
          }
        }
        n1545 = case shown="True" "Red Laser ON" {
          tunnel: "Laser interlacing mode" -> [_ w2206]
          tunnel: [enum32{"Laser ON", "Laser OFF", "Interlace"}."Laser OFF" ("Green laser mode") w2206] -> w2185
          tunnel: [FALSE w2202] -> w2184
          frame False {
          }
          frame True {
            n1546 = local read "Red FB On/Off"() -> (w2203:bool)
            n1547 = Equal?(x=w2206, y=enum32{"Laser ON", "Laser OFF", "Interlace"}."Interlace") -> (x = y?=w2204:bool)
            n1548 = And(x=w2204, y=w2203) -> (x .and. y?=w2202:bool)
          }
        }
        n1549 = case shown="True" "Blue Laser ON" {
          tunnel: "Laser interlacing mode" -> [_ w2197]
          tunnel: [enum32{"Laser ON", "Laser OFF", "Interlace"}."Laser OFF" ("Green laser mode") w2197] -> w2181
          tunnel: [FALSE w2195] -> w2180
          frame False {
          }
          frame True {
            n1550 = local read "Blue FB On/Off"() -> (w2196:bool)
            n1551 = Equal?(x=w2197, y=enum32{"Laser ON", "Laser OFF", "Interlace"}."Interlace") -> (x = y?=w2198:bool)
            n1552 = And(x=w2198, y=w2196) -> (x .and. y?=w2195:bool)
          }
        }
        n1553 = xnode "Read/Write Control"("FPGA VI Reference In"=w2192, "error in"=w2190, "Operating Mode"=w2189, "Operating Mode 2"=w2189, "Green FB On/Off"=w2188, "Red Laser Operating Mode"=w2185, "RI Operating Mode 2"=w2185, "Red FB On/Off"=w2184, "BI Operating Mode (AO)"=w2181, "Blue Laser Operating Mode (D)"=w2181, "Blue FB On/Off"=w2180) -> ("error out"=w2191:errorcluster)  [unwired: 1 out]
      }
      event "Invert laser interlacing": Value Change {
        n1554 = event-data() -> ()  [unwired: 7 out]
        n1555 = xnode "Read/Write Control"("FPGA VI Reference In"=w2217, "error in"=w2215, "Invert GI"="Invert laser interlacing", "Invert GI 2"="Invert laser interlacing", "Invert RI"="Invert laser interlacing", "Invert RI 2"="Invert laser interlacing", "Invert BI (AO)"="Invert laser interlacing", "Invert BI (D)"="Invert laser interlacing") -> ("error out"=w2216:errorcluster)  [unwired: 1 out]
      }
      event "Green FB Setpoint (mV)", "Green FB Gains", "Green FB On/Off", "Green Intensity % (FB OFF)", "Green int current ON count adj": Value Change {
        n1556 = event-data() -> ()  [unwired: 7 out]
        n1557 = local read "Green FB Setpoint (mV)"() -> (w2228:dbl)
        n1558 = Multiply(x=w2228, y=3.2767) -> (x*y=w2227:dbl)
        n1559 = local read "Green Intensity % (FB OFF)"() -> (w2231:dbl)
        n1560 = Multiply(x=w2231, y=655.35) -> (x*y=w2232:dbl)
        n1561 = To Unsigned Word Integer(number=w2232) -> (unsigned 16bit integer=w2230:u16)
        n1562 = local read "Green int current ON count adj"() -> (w2234:u32)
        n1563 = local read "Laser interlacing mode"() -> (w2224:enum32{"Laser ON", "Laser OFF", "Interlace"})
        n1564 = local read "Green FB Gains"() -> (w2221:T9)
        n1565 = local read "Green Laser ON"() -> (w2225:bool)
        n1566 = local read "Green FB On/Off"() -> (w2235:bool)
        n1567 = Equal?(x=w2224, y=enum32{"Laser ON", "Laser OFF", "Interlace"}."Interlace") -> (x = y?=w2222:bool)
        n1568 = Unbundle By Name(w2221) -> ("proportional gain (Kc)"=w2220:i16, "integral gain (Kc*Ts/Ti)"=w2219:i16, "derivative gain (Kc*Td/Ts)"=w2218:i16)
        n1569 = Compound Arithmetic op=AND(w2222, w2235, w2225) -> (w2226:bool)
        n1570 = xnode "Read/Write Control"("FPGA VI Reference In"=w2238, "error in"=w2237, "Green FB Setpoint"=w2227, "Green FB On/Off"=w2226, "Current Out"=w2230, "Green int current ON count adj"=w2234, "P3"=w2220, "I3"=w2219, "D3"=w2218) -> ("error out"=w2236:errorcluster)  [unwired: 1 out]
      }
      event "Blue FB Setpoint (mV)", "Blue FB Gains", "Blue FB On/Off", "Blue Intensity % (FB OFF)", "Blue int AO ON count adjust": Value Change {
        # "16 bit analog out"
        n1571 = event-data() -> ()  [unwired: 7 out]
        n1572 = Multiply(x="Blue FB Setpoint (mV)", y=3.2767) -> (x*y=w2252:dbl)
        n1573 = Multiply(x="Blue Intensity % (FB OFF)", y=655.35) -> (x*y=w2255:dbl)
        n1574 = To Unsigned Word Integer(number=w2255) -> (unsigned 16bit integer=w2254:u16)
        n1575 = local read "Laser interlacing mode"() -> (w2250:enum32{"Laser ON", "Laser OFF", "Interlace"})
        n1576 = Unbundle By Name("Blue FB Gains") -> ("proportional gain (Kc)"=w2247:i16, "integral gain (Kc*Ts/Ti)"=w2246:i16, "derivative gain (Kc*Td/Ts)"=w2245:i16)
        n1577 = local read "Blue Laser ON"() -> (w2239:bool)
        n1578 = Equal?(x=w2250, y=enum32{"Laser ON", "Laser OFF", "Interlace"}."Interlace") -> (x = y?=w2248:bool)
        n1579 = Compound Arithmetic op=AND(w2248, "Blue FB On/Off", w2239) -> (w2251:bool)
        n1580 = xnode "Read/Write Control"("FPGA VI Reference In"=w2259, "error in"=w2258, "Blue FB Setpoint"=w2252, "Blue FB On/Off"=w2251, "BI Current Out"=w2254, "Blue current ON count adj (AO)"="Blue int AO ON count adjust", "P5"=w2247, "I5"=w2246, "D5"=w2245) -> ("error out"=w2257:errorcluster)  [unwired: 1 out]
      }
      event "Red FB Setpoint (mV)", "Red FB Gains", "Red FB On/Off", "Red Intensity % (FB OFF)": Value Change {
        n1581 = event-data() -> ()  [unwired: 7 out]
        n1582 = local read "Red FB Setpoint (mV)"() -> (w2271:dbl)
        n1583 = Multiply(x=w2271, y=3.2767) -> (x*y=w2270:dbl)
        n1584 = local read "Red Intensity % (FB OFF)"() -> (w2260:dbl)
        n1585 = Multiply(x=w2260, y=655.35) -> (x*y=w2274:dbl)
        n1586 = To Unsigned Word Integer(number=w2274) -> (unsigned 16bit integer=w2273:u16)
        n1587 = local read "Laser interlacing mode"() -> (w2267:enum32{"Laser ON", "Laser OFF", "Interlace"})
        n1588 = local read "Red FB Gains"() -> (w2264:T9)